vi "Main.vi"() -> ()   [LabVIEW 2020] (continued)
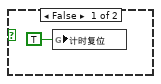
[diagram p2: hidden frame]
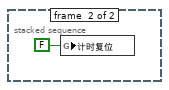
[diagram p3: hidden frame]
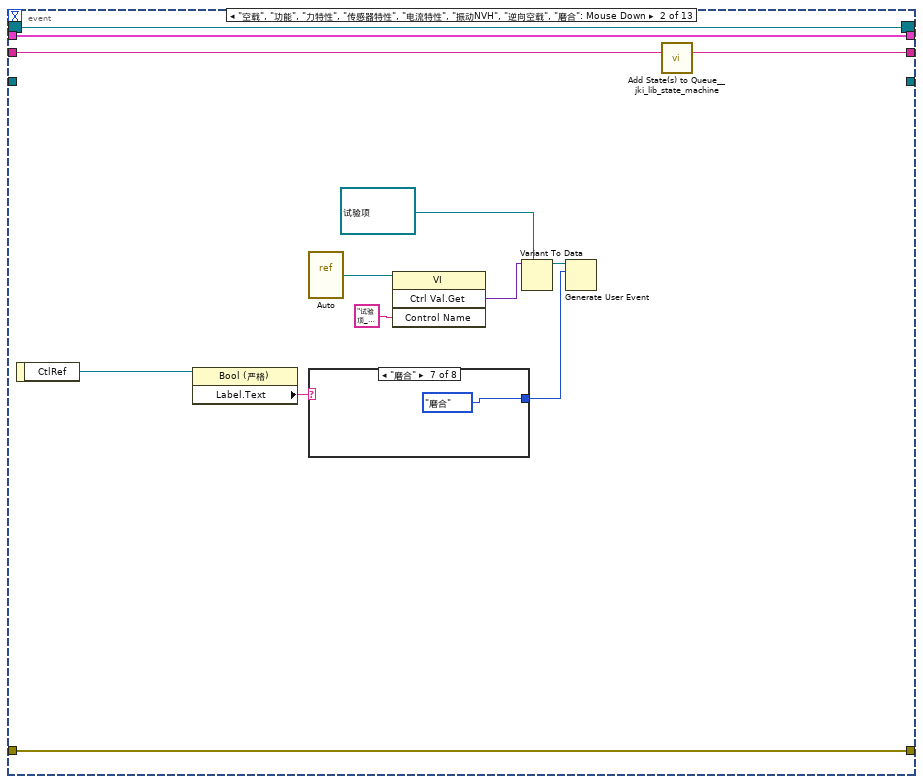
[diagram p4: hidden frame]
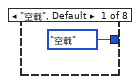
[diagram p5: hidden frame]
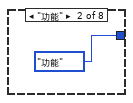
[diagram p6: hidden frame]
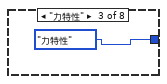
[diagram p7: hidden frame]
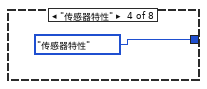
[diagram p8: hidden frame]
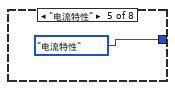
[diagram p9: hidden frame]
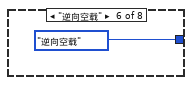
[diagram p10: hidden frame]
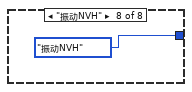
[diagram p11: hidden frame]
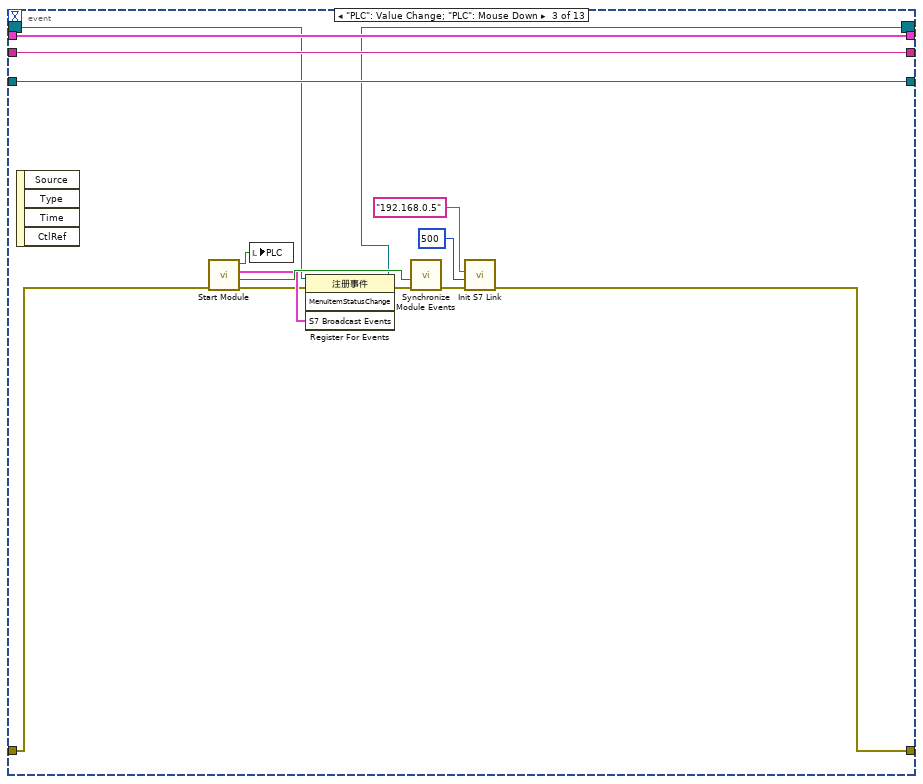
[diagram p12: hidden frame]
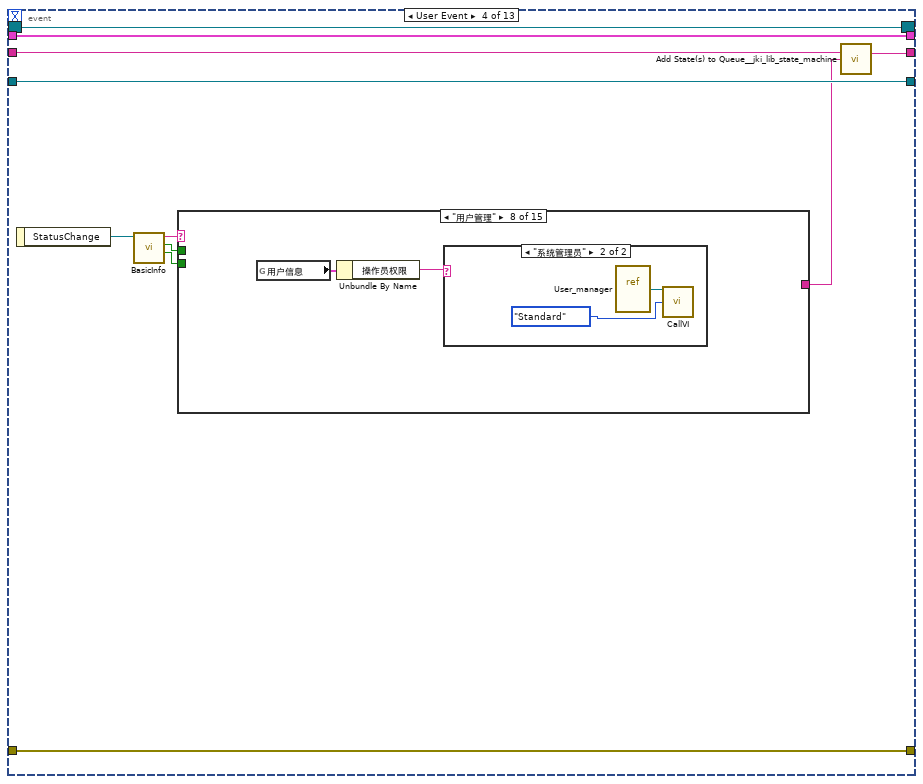
[diagram p13: hidden frame]
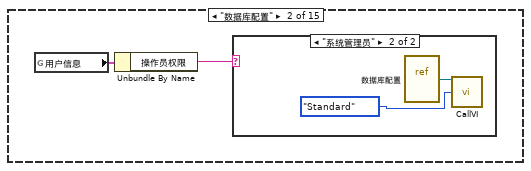
[diagram p15: hidden frame]
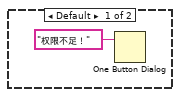
[diagram p16: hidden frame]
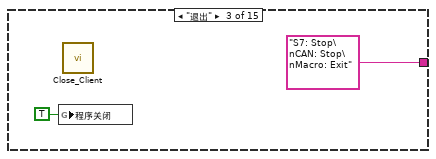
[diagram p17: hidden frame]
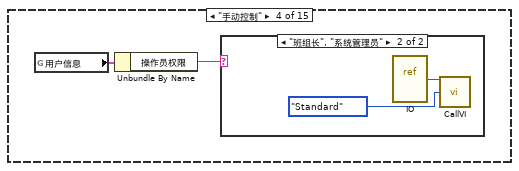
[diagram p18: hidden frame]
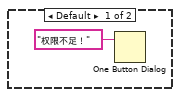
[diagram p19: hidden frame]
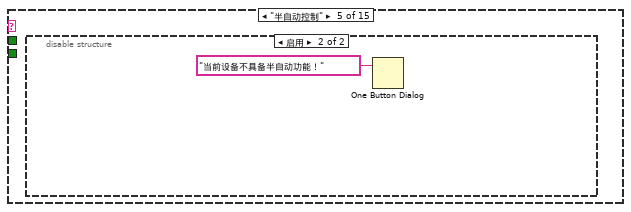
[diagram p20: hidden frame]
                  }
                  frame True {
                    n121 = vi-ref "Auto.vi"() -> (w205:refnum<vi>)
                    n122 = invoke class="VI" method="Ctrl Val.Set"(reference=w205, "Control Name"="STEP" ("控件名"), "Value"="退出自动" ("控件名")) -> ()  [unwired: 2 in, 5 out]
                  }
                }
              }
            }
            n123 = call <vilib>:"Add State(s) to Queue__jki_lib_state_machine.vi"("State(s) in (\"\")"=w192) -> ("States Out"=w193:string)  [unwired: 14 in]
          }
          event "错误": Mouse Down {
            n124 = event-data() -> ()  [unwired: 1 in, 8 out]
            n125 = vi-ref "报警信息.vi"() -> (w208:refnum<vi>)
            n126 = call "CallVI.vi"("VI引用"=w208, "状态"=T3."Standard") -> ()  [unwired: 12 in, 2 out]
            n127 = call <vilib>:"Add State(s) to Queue__jki_lib_state_machine.vi"("State(s) in (\"\")"=w210) -> ("States Out"=w211:string)  [unwired: 14 in]
          }
          event Panel Close? {
            n128 = event-data() -> ()  [unwired: 1 in, 1 out]
            n129 = disable-structure shown="禁用" {
              frame Disabled {
                n130 = call "Close.vi"() -> ()  [unwired: 11 in, 1 out]
              }
              frame Enabled {
              }
            }
            n131 = global write "Global.vi" "程序关闭"(TRUE ("程序关闭")) -> ()
            n132 = call <vilib>:"Add State(s) to Queue__jki_lib_state_machine.vi"("State(s) in Front (\"\")"="S7: Stop\nMacro: Exit", "State(s) in (\"\")"=w220) -> ("States Out"=w219:string)  [unwired: 13 in]
            n133 = event-data("Discard?"=TRUE) -> ()  [unwired: 1 in, 1 out]
          }
          event "更换产品": Value Change {
            n134 = event-data() -> ("NewVal"=w223:refnum<vi>)  [unwired: 1 in, 5 out]
            n135 = stacked-sequence {
              tunnel: w223 -> [w229]
              tunnel: [w228] -> w221
              frame #0 {
                n136 = stacked-sequence {
                  tunnel: w229 -> [w237 _ _]
                  tunnel: [_ w241 _] -> w228
                  frame #0 {
                    n137 = disable-structure shown="禁用" {
                      disable-tunnel: w237 -> [w239 _]
                      frame Disabled {
                        n138 = control-ref of="子面板"() -> (w238:refnum<vi>)
                        n139 = call "Call_SubPanal.vi"("VI引用句柄"=w239, "SubPnl引用句柄"=w238) -> ()  [unwired: 9 in, 1 out]
                      }
                      frame Enabled {
                      }
                    }
                    n140 = vi-ref "Auto.vi"() -> (w236:refnum<vi>)
                    n141 = invoke class="VI" method="Ctrl Val.Get"(reference=w236, "Control Name"="产品_EVENT" ("控件名")) -> ("Get Control Value Variant"=w235:variant)  [unwired: 2 in, 3 out]
                    n142 = global read "Global.vi" "产品型号"() -> (w231:string)
                    n143 = local write "产品型号"(w231) -> ()
                    n144 = Variant To Data(type=refnum<user-event> refnum ("产品_EVENT"), Variant=w235) -> (data=w232:refnum<user-event>, error out=w230:errorcluster)  [unwired: 1 in]
                    n145 = Generate User Event(user event=w232, event data cluster=w231, error in=w230) -> ()  [unwired: 1 in, 2 out]
                  }
                  frame #1 {
                    n146 = global read "Global.vi" "启用CAN"() -> (w240:bool)
                    n147 = case shown="真" w240 {
                      tunnel: ["CAN: Stop" "CAN: Stop"] -> w241
                      frame False {
                      }
                      frame True {
                        (unwired) "CAN: Stop\nIdle\nCAN: Start"
                      }
                    }
                  }
                  frame #2 {
                    n148 = control-ref of="磨合"() -> (w244:refnum<vi>)
                    n149 = control-ref of="空载"() -> (w249:refnum<vi>)
                    n150 = control-ref of="功能"() -> (w250:refnum<vi>)
                    n151 = control-ref of="力特性"() -> (w251:refnum<vi>)
                    n152 = control-ref of="电流特性"() -> (w248:refnum<vi>)
                    n153 = control-ref of="传感器特性"() -> (w247:refnum<vi>)
                    n154 = control-ref of="逆向空载"() -> (w246:refnum<vi>)
                    n155 = control-ref of="振动NVH"() -> (w245:refnum<vi>)
                    n156 = global read "Global.vi" "试验项目"() -> (w254:bool[])
                    n157 = Build Array(w249, w250, w251, w248, w247, w246, w245, w244) -> (w253:refnum<vi>[])
                    n158 = for {
                      tunnel: w253 -> [w258] mode=indexing
                      tunnel: w254 -> [w259] mode=indexing
                      shift-right: [w255] -> _
                      shift-left: 2095 -> [w256]
                      i -> [w257]
                      n159 = case shown="真" w259 {
                        tunnel: w258 -> [w260 w268]
                        tunnel: w257 -> [_ _]
                        tunnel: w256 -> [w262 w265]
                        tunnel: [w262 w263] -> w255
                        frame False {
                          n160 = property class="Bool (严格)"(reference=w260, "Top"=2000) -> ()  [unwired: 1 in, 2 out]
                        }
                        frame True {
                          n161 = Add(x=w265, y=115) -> (x+y=w263:i32)
                          n162 = Bundle(w263, 1300) -> (w266:cluster{i32, i32})  [unwired: 1 in]
                          n163 = property class="Bool (严格)"(reference=w268, "Position"=w266) -> ()  [unwired: 1 in, 2 out]
                        }
                      }
                    }
                  }
                }
              }
            }
            n164 = call <vilib>:"Add State(s) to Queue__jki_lib_state_machine.vi"("State(s) in Front (\"\")"=w221, "State(s) in (\"\")"=w224) -> ("States Out"=w225:string)  [unwired: 13 in]
          }
          event "Andon": Value Change {
            w279 = "最终性能试验台2" ("设备名称")
            n165 = event-data() -> ("NewVal"=w269:enum32{"未选择", "缺料报警", "质量报警", "故障报警"})  [unwired: 1 in]
            n166 = global read "用户信息.vi" "用户信息"() -> (w270:T6)
            n167 = Unbundle By Name(w270) -> ("操作员姓名"=w278:string)
            n168 = case shown="\"故障报警\"" w269 {
              tunnel: w279 -> [_ _ _ _]
              tunnel: w278 -> [_ _ _ _]
              tunnel: [enum16{"设备离线", "设备正常", "设备缺料", "设备故障", "质量报警"}."设备正常" ("设备状态") enum16{"设备离线", "设备正常", "设备缺料", "设备故障", "质量报警"}."设备缺料" ("设备状态") enum16{"设备离线", "设备正常", "设备缺料", "设备故障", "质量报警"}."质量报警" ("设备状态") enum16{"设备离线", "设备正常", "设备缺料", "设备故障", "质量报警"}."设备故障" ("设备状态")] -> w276
              frame "未选择", Default {
              }
              frame "缺料报警" {
              }
              frame "质量报警" {
              }
              frame "故障报警" {
              }
            }
            n169 = Bundle By Name(cluster=T4 {"设备名称"="", "操作人员"="", "设备状态"=enum."设备离线", "附加信息"=""} ("设备信息"), "设备名称"=w279, "操作人员"=w278, "设备状态"=w276) -> (w271:T4)
            n170 = call "Change_Client.vi"("设备信息"=w271) -> ()  [unwired: 10 in, 1 out]
          }
        }
      }
      frame "---------- Core ----------" {
        n171 = call <vilib>:"Add State(s) to Queue__jki_lib_state_machine.vi"("State(s) in (\"\")"=w289) -> ("States Out"=w288:string)  [unwired: 14 in]
      }
      frame Default {
        w301 = 42 items=["No error", "Argument error", "Memory is full", "Out of zone", "End of file", "File already open", "Generic file I/O error", "File not found", "File permission error", "Disk is full", "Duplicate path", "Too many files open", "System feature not enabled", "Resource file not found", "Cannot add resource", "Resource not found", "Image not found", "Image memory error", "Pen does not exist", "Config type invalid", "Config token not found", "Config parse error", "Config memory error", "Bad external code format", "Bad external code offset", "External code not present", "Null window", "Destroy window error", "Null menu", "Print aborted", "Bad print record", "Print driver error", "Windows error during printing", "Memory error during printing", "Print dialog error", "Generic print error", "Invalid device refnum", "Device not found", "Device parameter error", "Device unit error", "Cannot open device", "Device call aborted", "Generic error", "Cancelled by user", "Object ID too low", "Object ID too high", "Object not in heap", "Unknown heap", "Unknown object (invalid DefProc)", "Unknown object (DefProc not in table)", "Message out of range", "Invalid (null) method", "Unknown message", "Manager call not supported", "Bad address", "Network operation in progress", "Network operation timed out", "Connection is busy", "Network attribute not supported", "Network error", "Address in use", "System out of memory", "Connection aborted", "Connection refused", "Not connected", "Already connected", "Connection closed", "Initialization error (interapplication manager)", "Bad occurrence", "Wait on unbound occurrence handler", "Occurrence queue overflow", "Datalog type conflict", "Unused", "Unrecognized type (interapplication manager)", "Memory corrupt", "Failed to make temporary DLL", "Old CIN version", "Drag socket not found", "Failed to load drop-object", "Failed to register OLE object", "Failed to release OLE object", "Format specifier type mismatch", "Unknown format specifier", "Too few format specifiers", "Too many format specifiers", "Scan failed", "Newer CIN version", "Error converting to variant", "Runtime menu error", "Password tampered", "Variant attribute not found", "Incompatible variant data type", "Event data is not available", "Event Store is not present", "Occurrence is not found", "Event Queue is not created", "Event info is not available", "Refnum passed is NULL", "Error retrieving Class GUID", "Error retrieving CoClass GUID", "Error retrieving TypeLib GUID.", "Bad built application magic bytes.", "Specific driver is different from the specific driver associated with the Logical Name.", "There is no session opened to the class driver.", "Max Error", "MAX - Error with config objects", "MAX - Error loading configuration", "MAX - Group not supported"]
        # "Current State"
        n172 = Format Into String(format string="Software Exception: Unhandled State \"%s\"." ("message"), error in=w297, w292) -> (resulting string=w300:string, error out=w299:errorcluster)  [unwired: 1 in]
        n173 = call <vilib>:"Error Cluster From Error Code.vi"("show call chain? (False)"=TRUE, "error in (no error)"=w299, "error message (\"\")"=w300, "error code (0)"=w301) -> ("error out"=w298:errorcluster)  [unwired: 5 in]
        n174 = call <vilib>:"Add State(s) to Queue__jki_lib_state_machine.vi"("State(s) in (\"\")"=w296) -> ("States Out"=w295:string)  [unwired: 14 in]
      }
      frame "Initialize Core Data" {
        # "originally closed?"
        # "exe?"
        n175 = property class="VI"() -> ("Front Panel.Open"=w312:bool)  [unwired: 2 in, 2 out]
        n176 = property class="App"() -> ("App.Kind"=w311:T5)  [unwired: 2 in, 2 out]
        n177 = control-ref of="Current VI Reference"() -> (w305:refnum<vi>)
        n178 = Not(x=w312) -> (.not. x?=w309:bool)
        n179 = Equal?(x=w311, y=T5."Run Time System" ("Application:Kind")) -> (x = y?=w308:bool)
        n180 = Or(x=w309, y=w308) -> (x .or. y?=w306:bool)
        n181 = Bundle By Name(cluster=w307, "Core.Current VI Reference"=w305, "Core.Close Panel on Exit?"=w306) -> (w314:T7)
        n182 = call <vilib>:"Add State(s) to Queue__jki_lib_state_machine.vi"("State(s) in (\"\")"=w316) -> ("States Out"=w315:string)  [unwired: 14 in]
      }
      frame "Error Handler" {
        n183 = call <vilib>:"General Error Handler.vi"("error in (no error)"=w320) -> ()  [unwired: 10 in, 5 out]
        n184 = call <vilib>:"Add State(s) to Queue__jki_lib_state_machine.vi"("State(s) in Front (\"\")"="/* Post Error States", "State(s) in (\"\")"=w324) -> ("States Out"=w323:string)  [unwired: 13 in]
      }
      frame "Exit" {
        n185 = Quit LabVIEW(quit? (T)=TRUE ("退出？(T)")) -> ()
        n186 = call <vilib>:"Add State(s) to Queue__jki_lib_state_machine.vi"("State(s) in (\"\")"=w332) -> ("States Out"=w331:string)  [unwired: 14 in]
      }
      frame "--------- Library --------" {
        n187 = call <vilib>:"Add State(s) to Queue__jki_lib_state_machine.vi"("State(s) in (\"\")"=w338) -> ("States Out"=w337:string)  [unwired: 14 in]
      }
      frame "S7: Initialize" {
        n188 = property on="PLC" class="Bool (严格)"("Val(Sgnl)"=FALSE ("值(信号)")) -> ()  [unwired: 2 in, 2 out]
      }
      frame "S7: Stop" {
        n189 = call "Stop Module.vi"("error in (no error)"=w347) -> ("error out"=w346:errorcluster)  [unwired: 10 in]
        n190 = call <vilib>:"Add State(s) to Queue__jki_lib_state_machine.vi"("State(s) in (\"\")"=w348) -> ("States Out"=w349:string)  [unwired: 14 in]
      }
      frame "CAN: Start" {
        n191 = disable-structure shown="禁用" {
          frame Enabled {
            n192 = while {
              stop <- w358 stop-if-true
              n193 = vi-ref "CAN.vi"() -> (w363:refnum<vi>)
              n194 = call "CallVI.vi"("VI引用"=w363, "状态"=T3."Hidden") -> ("VI引用OUT"=w361:refnum<vi>, "错误输出"=w360:errorcluster)  [unwired: 12 in]
              n195 = property class="VI"(reference=w361, error in=w360) -> ("Exec.State"=w359:T8)  [unwired: 2 out]
              n196 = case shown="\"Bad\", 默认" w359 {
                tunnel: [w367 TRUE TRUE] -> w358
                frame "Bad", Default {
                  n197 = Two Button Dialog(message="CAN卡打开失败！" ("消息"), 1:"重试" ("F按钮名称（“取消”）"), 2:"忽略" ("T按钮名称（“确定”）")) -> (T button?=w367:bool)
                }
                frame "Run top level" {
                }
                frame "Running" {
                }
              }
            }
          }
          frame Disabled {
            n198 = call "CAN_Start.vi"() -> ("Success"=→"CAN":bool)  [unwired: 11 in]
          }
        }
        n199 = call <vilib>:"Add State(s) to Queue__jki_lib_state_machine.vi"("State(s) in (\"\")"=w354) -> ("States Out"=w355:string)  [unwired: 14 in]
      }
      frame "CAN: Stop" {
        n200 = disable-structure shown="启用" {
          frame Enabled {
            n201 = vi-ref "CAN.vi"() -> (w379:refnum<vi>)
            n202 = invoke class="VI" method="Ctrl Val.Set"(reference=w379, "Control Name"="Stop" ("控件名"), "Value"=TRUE) -> ()  [unwired: 2 in, 5 out]
          }
          frame Disabled {
            n203 = call "CAN_Stop.vi"() -> ()  [unwired: 12 in]
            n204 = local write "CAN"(FALSE ("CAN")) -> ()
          }
        }
        n205 = call <vilib>:"Add State(s) to Queue__jki_lib_state_machine.vi"("State(s) in (\"\")"=w373) -> ("States Out"=w374:string)  [unwired: 14 in]
      }
      frame "---------- Data ----------" {
        n206 = call <vilib>:"Add State(s) to Queue__jki_lib_state_machine.vi"("State(s) in (\"\")"=w386) -> ("States Out"=w385:string)  [unwired: 14 in]
      }
      frame "Data: Initialize" {
        w392 = T9 {"Current VI Reference"=refnum, "Close Panel on Exit?"=FALSE}  # Core
        w394 = TRUE  # Your Boolean data
        w393 = ""  # Your string data
        n207 = control-ref of="CAN"() -> (w387:refnum<vi>)
        n208 = global write "Global.vi" "程序关闭"(FALSE ("程序关闭")) -> ()
        n209 = global write "Global.vi" "计时开始"(FALSE ("计时结束")) -> ()
        n210 = global write "Global.vi" "CAN"(w387) -> ()
        n211 = Bundle("Core"=w392, "Your Boolean data"=w394, "Your string data"=w393) -> (w396:T7)  [unwired: 1 in]
        n212 = call <vilib>:"Add State(s) to Queue__jki_lib_state_machine.vi"("State(s) in (\"\")"=w398) -> ("States Out"=w397:string)  [unwired: 14 in]
      }
      frame "Data: Cleanup" {
        n213 = Unbundle By Name(w401) -> ("Core.Current VI Reference"=w404:refnum<vi>)
        n214 = Close Reference(reference=w404, error in (no error)=w403) -> (error out=w402:errorcluster)
        n215 = call <vilib>:"Add State(s) to Queue__jki_lib_state_machine.vi"("State(s) in (\"\")"=w406) -> ("States Out"=w405:string)  [unwired: 14 in]
      }
      frame "---------- UI ----------" {
        # "Do not put any code in this frame.\n(It is a separator no-op. You can make a copy of this frame to create a new UI frame)"
        n216 = call <vilib>:"Add State(s) to Queue__jki_lib_state_machine.vi"("State(s) in (\"\")"=w412) -> ("States Out"=w411:string)  [unwired: 14 in]
      }
      frame "UI: Initialize" {
        n217 = disable-structure shown="启用" {
          disable-tunnel: [w426 _] -> w416
          disable-tunnel: w413 -> [w424 _]
          frame Enabled {
            n218 = vi-ref "Auto.vi"() -> (w425:refnum<vi>)
            n219 = property class="VI"(reference=w425) -> (reference out=w423:refnum<vi>, "FP.State"=w422:T3)  [unwired: 1 in, 1 out]
            n220 = case shown="\"Invalid\", \"Closed\"" w422 {
              tunnel: w424 -> [w432 w434]
              tunnel: w423 -> [w433 w435]
              tunnel: [w431 w435] -> w420
              tunnel: [w430 w434] -> w421
              frame "Standard", Default {
                n221 = invoke class="VI" method="FP.Close"(reference=w433, error in=w432) -> (reference out=w431:refnum<vi>, error out=w430:errorcluster)  [unwired: 1 in, 1 out]
              }
              frame "Invalid", "Closed" {
              }
            }
            n222 = invoke on="子面板" class="SubPnl" method="Insert VI"(error in=w421, "VI Ref"=w420) -> (error out=w429:errorcluster)  [unwired: 2 in, 3 out]
            n223 = invoke class="VI" method="Run VI"(reference=w420, error in=w429, "Wait until done"=FALSE ("结束前等待"), "Auto Dispose Ref"=TRUE ("自动销毁引用")) -> (error out=w426:errorcluster)  [unwired: 1 in, 4 out]
          }
          frame Disabled {
            n224 = vi-ref "Auto.vi"() -> (w437:refnum<vi>)
            n225 = call "CallVI.vi"("VI引用"=w437, "状态"=T3."Maximized") -> ()  [unwired: 12 in, 2 out]
          }
        }
        n226 = call <vilib>:"Add State(s) to Queue__jki_lib_state_machine.vi"("State(s) in (\"\")"=w419) -> ("States Out"=w418:string)  [unwired: 14 in]
      }
      frame "UI: Init" {
        n227 = stacked-sequence {
          tunnel: w439 -> [_ _ _ _ _]
          frame #0 {
            n228 = disable-structure shown="禁用" {
              frame Disabled {
                n229 = call "Open.vi"() -> ()  [unwired: 11 in, 1 out]
              }
              frame Enabled {
              }
            }
          }
          frame #1 {
            n230 = global write "Global.vi" "程序关闭"(FALSE ("程序关闭")) -> ()
            n231 = control-ref of="电流特性"() -> (w448:refnum<vi>)
            n232 = control-ref of="空载"() -> (w451:refnum<vi>)
            n233 = control-ref of="力特性"() -> (w449:refnum<vi>)
            n234 = control-ref of="功能"() -> (w450:refnum<vi>)
            n235 = global write "A180648.vi" "LED-电流特性"(w448) -> ()
            n236 = global write "A180648.vi" "LED-空载"(w451) -> ()
            n237 = global write "A180648.vi" "LED-力特性"(w449) -> ()
            n238 = global write "A180648.vi" "LED-功能"(w450) -> ()
            n239 = control-ref of="逆向空载"() -> (w447:refnum<vi>)
            n240 = control-ref of="振动NVH"() -> (w445:refnum<vi>)
            n241 = control-ref of="磨合"() -> (w444:refnum<vi>)
            n242 = control-ref of="传感器特性"() -> (w446:refnum<vi>)
            n243 = global write "A180648.vi" "LED-传感器特性"(w446) -> ()
            n244 = global write "A180648.vi" "LED-逆向空载"(w447) -> ()
            n245 = global write "A180648.vi" "LED-振动NVH"(w445) -> ()
            n246 = global write "A180648.vi" "LED-磨合"(w444) -> ()
          }
          frame #2 {
            w459 = 0
            n247 = shared-variable "我的电脑\\Global.lvlib\\总成追溯码"("   " ("工位追溯码")) -> ()  [unwired: 1 in, 1 out]
            n248 = global write "Global.vi" "生产数量"(w459) -> ()
            n249 = global write "Global.vi" "合格数量"(w459) -> ()
            n250 = global read "Global.vi" "用户信息"() -> (w456:T10)
            n251 = global read "Global.vi" "联机模式"() -> (w453:enum16{"单机", "追溯"})
            n252 = Unbundle By Name(w456) -> ("用户名"=→"userName":string, "用户权限"=→"userStatus":string)
            n253 = case shown="\"追溯\"" w453 {
              tunnel: ["联网" ("connectionMode") "单机" ("connectionMode")] -> w460
              frame "追溯" {
              }
              frame "单机", Default {
              }
            }
            "connectionMode" <- w460
            "产品型号" <- "" ("产品型号")
          }
          frame #3 {
            n254 = control-ref of="提示信息"() -> (w465:refnum<vi>)
            n255 = control-ref of="自动"() -> (w466:refnum<vi>)
            n256 = control-ref of="错误"() -> (w467:refnum<vi>)
            n257 = control-ref of="Result"() -> (w468:refnum<vi>)
            n258 = control-ref of="更换产品"() -> (w464:refnum<vi>)
            n259 = global write "Global.vi" "提示信息"(w465) -> ()
            n260 = global write "Global.vi" "程序自动"(w466) -> ()
            n261 = global write "Global.vi" "报警图标"(w467) -> ()
            n262 = global write "Global.vi" "Result"(w468) -> ()
            n263 = global write "Global.vi" "更换产品"(w464) -> ()
            n264 = control-ref of="条码状态"() -> (w463:refnum<vi>)
            n265 = global write "Global.vi" "条码状态"(w463) -> ()
          }
          frame #4 {
            n266 = global read "Global.vi" "Result"() -> (w471:refnum<vi>)
            n267 = property class="Tbl"(reference=w471, "Row Headers[]"=string[] [], "Value"=string[][] []) -> ()  [unwired: 1 in, 2 out]
            n268 = call "Start_Client.vi"() -> ()  [unwired: 12 in]
          }
        }
        n269 = call <vilib>:"Add State(s) to Queue__jki_lib_state_machine.vi"("State(s) in (\"\")"=w443) -> ("States Out"=w442:string)  [unwired: 14 in]
      }
      frame "UI: Config" {
        n270 = vi-ref "Config.vi"() -> (w474:refnum<vi>)
        n271 = call "CallVI.vi"("VI引用"=w474, "状态"=T3."Standard") -> ()  [unwired: 12 in, 2 out]
        n272 = call <vilib>:"Add State(s) to Queue__jki_lib_state_machine.vi"("State(s) in (\"\")"=w479) -> ("States Out"=w478:string)  [unwired: 14 in]
      }
      frame "UI: Cursor Set" {
        # "Argument"
        n273 = case shown="\"Idle\", 默认" w482 {
          tunnel: w484 -> [w489 w491]
          tunnel: [w488 w490] -> w483
          frame "Idle", Default {
            n274 = call <vilib>:"Unset Busy.vi"("error in (no error)"=w489) -> ("error out"=w488:errorcluster)  [unwired: 10 in]
          }
          frame "Busy" {
            n275 = call <vilib>:"Set Busy.vi"("error in (no error)"=w491) -> ("error out"=w490:errorcluster)  [unwired: 9 in, 1 out]
          }
        }
        n276 = call <vilib>:"Add State(s) to Queue__jki_lib_state_machine.vi"("State(s) in (\"\")"=w487) -> ("States Out"=w486:string)  [unwired: 14 in]
      }
      frame "UI: Front Panel State" {
        # "Argument"
        n277 = Unbundle By Name(w496) -> ("Core.Current VI Reference"=w495:refnum<vi>)
        n278 = case shown="\"Close\"" w494 {
          tunnel: w498 -> [w504 w517]
          tunnel: [w506 w518] -> w497
          tunnel: w495 -> [w505 w515]
          frame "Open", Default {
            n279 = property class="VI"(reference=w505, error in=w504) -> (reference out=w502:refnum<vi>, error out=w503:errorcluster, "Front Panel.Open"=w501:bool)
            n280 = case shown="假" w501 {
              tunnel: [w509 w512] -> w506
              tunnel: w503 -> [w508 w512]
              tunnel: w502 -> [w507 _]
              frame False {
                n281 = invoke class="VI" method="FP.Open"(reference=w507, error in=w508, "Activate"=TRUE, "State"=T3."Standard") -> (error out=w509:errorcluster)  [unwired: 1 in, 4 out]
              }
              frame True {
              }
            }
          }
          frame "Close" {
            n282 = property class="VI"(reference=w515, error in=w517) -> (reference out=w514:refnum<vi>, error out=w516:errorcluster, "Front Panel.Open"=w513:bool)
            n283 = case shown="真" w513 {
              tunnel: [w519 w522] -> w518
              tunnel: w516 -> [w519 w521]
              tunnel: w514 -> [_ w520]
              frame False {
              }
              frame True {
                n284 = invoke class="VI" method="FP.Close"(reference=w520, error in=w521) -> (error out=w522:errorcluster)  [unwired: 1 in, 2 out]
              }
            }
          }
        }
        n285 = call <vilib>:"Add State(s) to Queue__jki_lib_state_machine.vi"("State(s) in (\"\")"=w500) -> ("States Out"=w499:string)  [unwired: 14 in]
      }
      frame "---------- Macro ----------" {
        n286 = call <vilib>:"Add State(s) to Queue__jki_lib_state_machine.vi"("State(s) in (\"\")"=w528) -> ("States Out"=w527:string)  [unwired: 14 in]
      }
      frame "Macro: Initialize" {
        n287 = call <vilib>:"Add State(s) to Queue__jki_lib_state_machine.vi"("State(s) in Front (\"\")"="Data: Initialize\nInitialize Core Data\nS7: Initialize\nIdle\nUI: Init\nUI: Front Panel State >> Open\nUI: Initialize\nUI: Config", "State(s) in (\"\")"=w535) -> ("States Out"=w534:string)  [unwired: 13 in]
      }
      frame "Macro: Exit" {
        n288 = Unbundle By Name(w544) -> ("Core.Close Panel on Exit?"=w543:bool)
        n289 = Select(t="UI: Front Panel State >> Close", s=w543, f="") -> (s? t:f=w540:string)
        n290 = call <vilib>:"Add State(s) to Queue__jki_lib_state_machine.vi"("State(s) in (\"\")"=w540, "State(s) at Back (\"\")"="Data: Cleanup\nExit") -> ("States Out"=w538:string)  [unwired: 13 in]
        n291 = call <vilib>:"Add State(s) to Queue__jki_lib_state_machine.vi"("State(s) in Front (\"\")"=w538, "State(s) in (\"\")"=w547) -> ("States Out"=w546:string)  [unwired: 13 in]
      }
    }
  }
  n292 = call-dynamic "Cleanup.vi"("MenuStrip in"=w6) -> ()  [unwired: 10 in, 1 out]
